vi "Measure DC 120629.vi"() -> ()   [LabVIEW 2011] (continued)
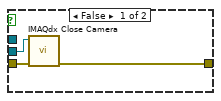
[diagram p3: hidden frame]
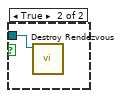
[diagram p7: hidden frame]
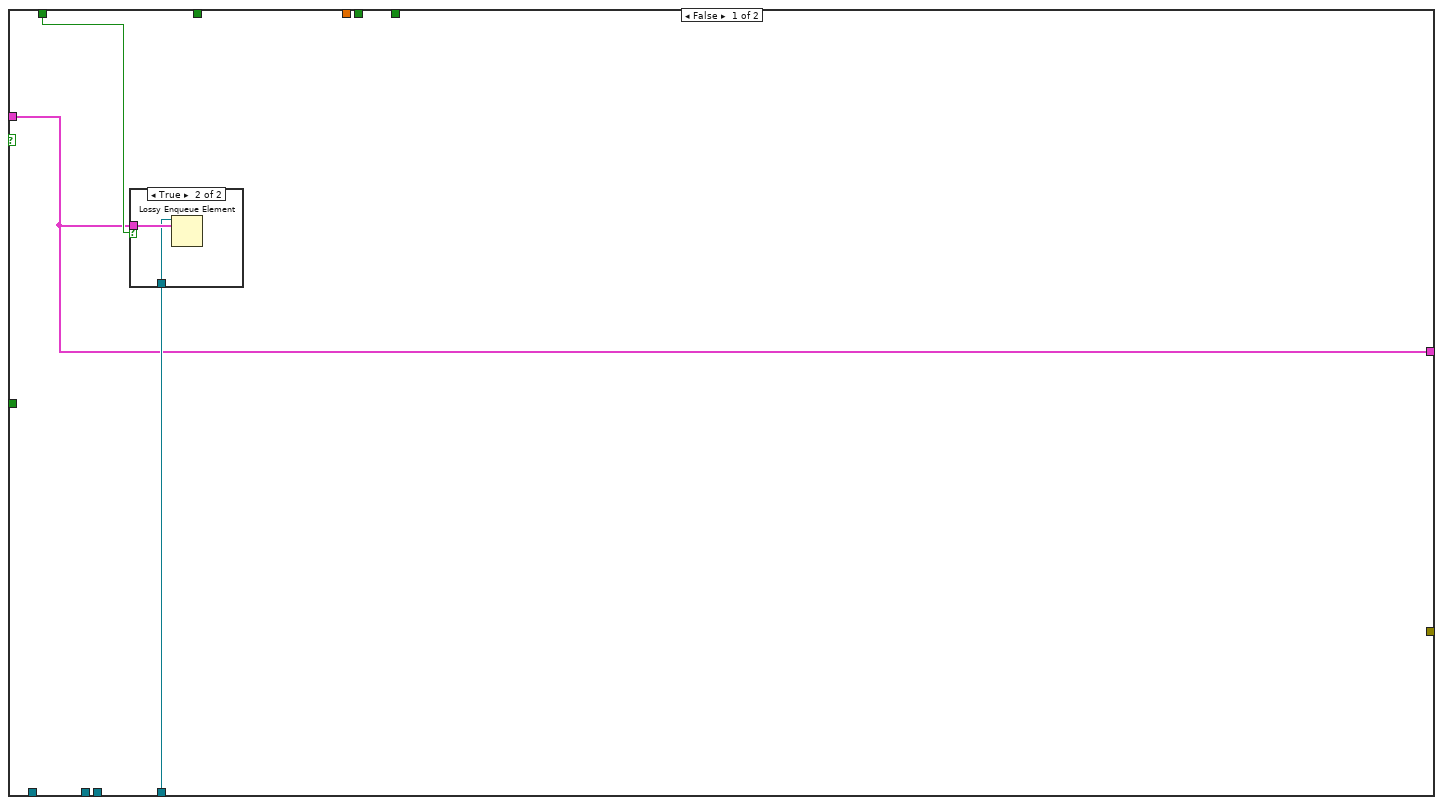
[diagram p10: hidden frame]
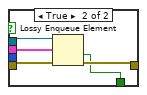
[diagram p13: hidden frame]
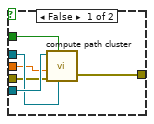
[diagram p17: hidden frame]
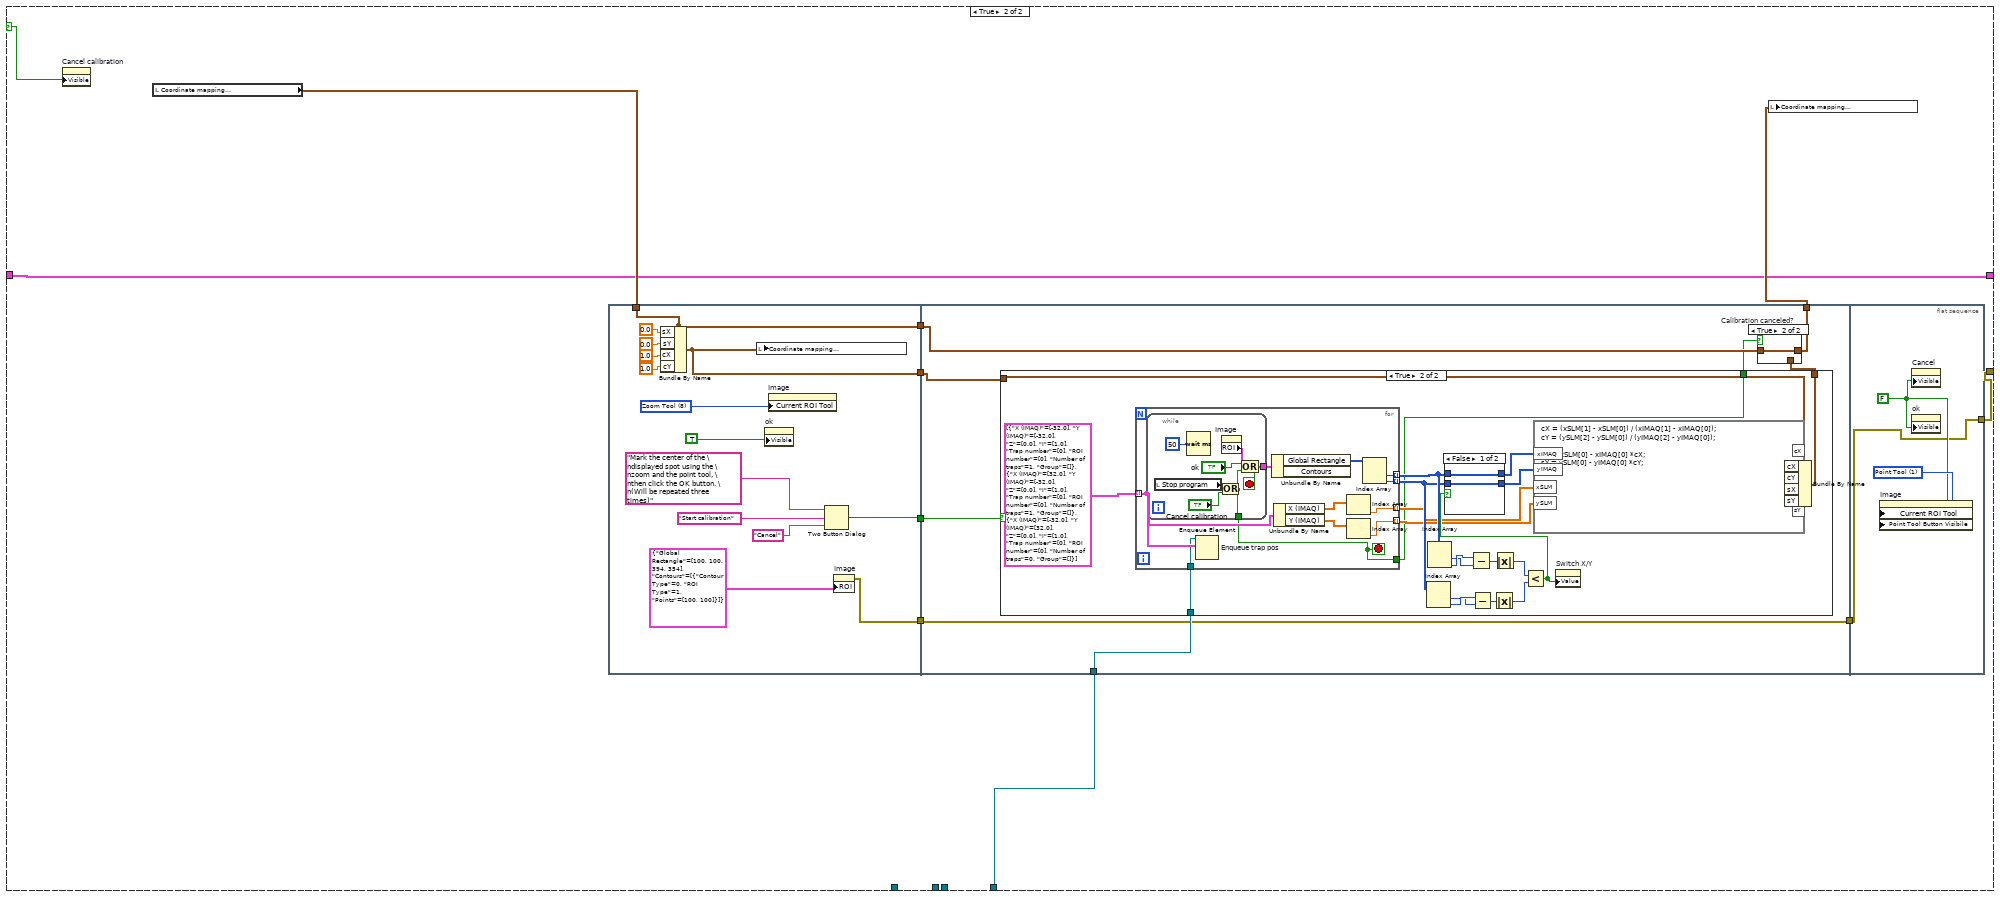
[diagram p18: hidden frame]
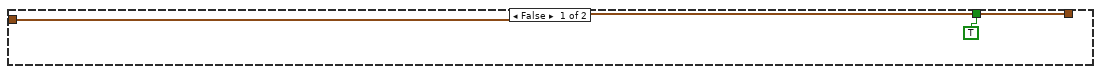
[diagram p20: hidden frame]
        tunnel: w280 -> [_ w301]
        tunnel: w284 -> [_ w300]
        frame False {
        }
        frame True {
          n112 = case shown="True" w305 {
            tunnel: w312 -> [w320 w331]
            tunnel: [w318 w330] -> w310
            tunnel: [w317 w329] -> w309
            tunnel: w311 -> [w318 w328]
            tunnel: [w319 w327] -> w308
            tunnel: [w314 w326] -> w303
            tunnel: [w316 w325] -> w307
            tunnel: w306 -> [w315 w325]
            tunnel: w304 -> [w313 w324]
            tunnel: w302 -> [_ w323]
            tunnel: w301 -> [_ w322]
            tunnel: w300 -> [_ w321]
            frame False {
              n113 = call <vilib>:"IMAQdx Grab.vi"("error in"=w313, "Image In"=w320, "Session In"=w315) -> ("error out"=w317:errorcluster, "Buffer Number Out"=w314:u32, "Image Out"=w319:T2, "Session Out"=w316:T9)  [unwired: 5 in]
            }
            frame True {
              n114 = case shown="True" w323 {
                tunnel: w331 -> [w338 _]
                tunnel: [w337 w346] -> w330
                tunnel: [w336 w348] -> w329
                tunnel: w328 -> [w335 w343]
                tunnel: [w334 w347] -> w327
                tunnel: [w333 w345] -> w326
                tunnel: w324 -> [w332 w344]
                tunnel: w322 -> [_ w340]
                tunnel: w321 -> [_ w339]
                frame False {
                  n115 = call <vilib>:"IMAQ Grab Acquire.vi"("error in (no error)"=w332, "Image In"=w338, "IMAQ Session In"=w335) -> ("error out"=w336:errorcluster, "Acquired Buffer Number"=w333:u32, "Image Out"=w334:T2, "IMAQ Session Out"=w337:refnum<k11>)  [unwired: 1 in, 4 out]
                }
                frame True {
                  n116 = case shown="True" w339 {
                    tunnel: w344 -> [w352 w353]
                    tunnel: w343 -> [w351 _]
                    tunnel: [w350 w353] -> w342
                    tunnel: [w349 w354] -> w341
                    tunnel: w340 -> [_ w354]
                    frame False {
                      n117 = property class="IMAQ"(reference=w351, error in=w352) -> (error out=w350:errorcluster, "Last Valid Frame"=w349:u32)  [unwired: 1 out]
                    }
                    frame True {
                    }
                  }
                  n118 = call <vilib>:"IMAQ Extract Buffer.vi"("error in (no error)"=w342, "Buffer to extract"=w341, "IMAQ Session In"=w343) -> ("error out"=w348:errorcluster, "Buffer Number"=w345:i32, "Image Out"=w347:T2, "IMAQ Session Out"=w346:refnum<k11>)  [unwired: 3 in, 2 out]
                }
              }
            }
          }
        }
      }
      n119 = call "IMAQ Cast Image"("Image Type"=w276, "Image Dst"=w275, "Image Src"=w278) -> ("Image Dst Out"=w273:T2)  [unwired: 7 in, 1 out]
      n120 = call "IMAQ Add"("Image Src A"=w274, "Image Src B"=w273) -> ("Image Dst Out"=w277:T2)  [unwired: 5 in, 1 out]
    }
    n121 = property class="IMAQ"(reference=w235) -> (reference out=w237:refnum<k11>, "Lost Frames"=→"Lost Frames":u32)  [unwired: 1 in, 1 out]
    n122 = call "IMAQ Divide"("Image Src A"=w221, "Constant"="Image\naveraging") -> ("Image Dst Out"=w217:T2)  [unwired: 5 in, 1 out]
    n123 = case shown="False" "?" {
      tunnel: w217 -> [w265 w272]
      tunnel: w216 -> [w264 w271]
      tunnel: [w263 w270] -> w215
      tunnel: "?" -> [w262 _]
      frame False {
        n124 = case shown="True" w262 {
          tunnel: w265 -> [w266 w269]
          tunnel: w264 -> [_ w268]
          tunnel: [w266 w267] -> w263
          frame False {
          }
          frame True {
            n125 = call "IMAQ Subtract"("Image Src A"=w269, "Image Src B"=w268) -> ("Image Dst Out"=w267:T2)  [unwired: 5 in, 1 out]
          }
        }
      }
      frame True {
        n126 = call "IMAQ Copy"("Image Dst"=w271, "Image Src"=w272) -> ("Image Dst Out"=w270:T2)  [unwired: 4 in, 1 out]
      }
    }
    n127 = case shown="True" "?" {
      tunnel: w215 -> [w355 w356]
      tunnel: [w355 w363] -> w228
      tunnel: w209 -> [_ w358]
      frame False {
      }
      frame True {
        w359 = T7 0 items=["Grayscale (U8)", "Grayscale (I16)", "Grayscale (SGL)", "Complex (CSG)", "RGB (U32)", "HSL (U32)", "RGB (U64)", "Grayscale (U16)"] ("Image Type")
        n128 = call "File Dialog"("start path"="start path") -> ("selected path"=w362:path, "cancelled"=w361:bool)  [unwired: 11 in, 2 out]
        n129 = call "IMAQ Cast Image"("Image Type"=w359, "Image Dst"=w358, "Image Src"=w356) -> ("Image Dst Out"=w357:T2)  [unwired: 7 in, 1 out]
        n130 = case shown="False" w361 {
          tunnel: [w364 w367] -> w363
          tunnel: w362 -> [w366 _]
          tunnel: w357 -> [w365 _]
          tunnel: w356 -> [w364 w367]
          frame False {
            n131 = call-poly "IMAQ Write File 2"("File Path"=w366, "Image"=w365) -> ()  [unwired: 8 in, 2 out]
          }
          frame True {
          }
        }
      }
    }
    n132 = call "IMAQ Quantify 2"("Image"=w228) -> ("Global Report"=→"Global Report":T3)  [unwired: 8 in, 2 out]
    n133 = case shown="True" "threshold" {
      tunnel: w228 -> [w368 w375]
      tunnel: [w368 w373] -> w233
      frame False {
      }
      frame True {
        n134 = Unbundle By Name("Range") -> ("Lower value"=w370:sgl)
        n135 = Select(t=w370, s="s", f=sgl 0.0) -> (s? t:f=w378:sgl)
        n136 = Select(t=sgl 0.0 ("Lower value"), s="s", f=w370) -> (s? t:f=w372:sgl)
        n137 = Bundle By Name(cluster="Range", "Lower value"=w372) -> (w376:cluster{"Lower value":sgl, "Upper value":sgl})
        n138 = call "IMAQ Subtract"("Image Src A"=w375, "Constant"=w378) -> ("Image Dst Out"=w374:T2)  [unwired: 5 in, 1 out]
        n139 = call "IMAQ Threshold"("Keep/Replace Value (Replace)"=FALSE, "Range"=w376, "Image Src"=w374) -> ("Image Dst Out"=w373:T2)  [unwired: 7 in, 1 out]
      }
    }
    n140 = case shown="True" "Video tracking" {
      tunnel: w233 -> [w388 w412]
      tunnel: w253 -> [_ w422]
      tunnel: w257 -> [w397 w421]
      tunnel: w245 -> [_ w420]
      tunnel: [w397 w419] -> w244
      tunnel: [_ w418] -> w242
      tunnel: [w381 w398] -> w256
      tunnel: w255 -> [w396 w417]
      tunnel: [w396 w416] -> w241
      tunnel: w248 -> [w393 _]
      tunnel: w249 -> [w392 w414]
      tunnel: "Display path" -> [w390 _]
      tunnel: [w387 w412] -> w232
      tunnel: [FALSE ("timed out?") w410] -> w230
      tunnel: "?" -> [_ w409]
      tunnel: w224 -> [w384 w403]
      tunnel: [w383 w400] -> _
      tunnel: "Switch X/Y" -> [w382 w399]
      tunnel: "ROI size" -> [w381 w398]
      frame False {
        n141 = Get Queue Status(queue=w393, return elements? (F)=w390) -> (elements=w394:T4[])  [unwired: 1 in, 7 out]
        n142 = Preview Queue Element(queue=w392, timeout in ms (-1)=10) -> (element=w391:T4)  [unwired: 1 in, 3 out]
        n143 = call "Create trap overlay.vi"("Current trap cluster"=w391, "Image in"=w388, "ROI size"=w381, "Switch X/Y"=w382, "Path"=w394) -> ("Image Out"=w387:T2)
        n144 = Wait (ms)(milliseconds to wait=u32 100) -> ()  [unwired: 1 out]
        n145 = call <vilib>:"Wait at Rendezvous.vi"("ms timeout (-1)"=0, "rendezvous"=w384) -> ("error out"=w383:errorcluster)  [unwired: 3 in, 2 out]
      }
      frame True {
        n146 = Preview Queue Element(queue=w414) -> (element=w415:T4)  [unwired: 2 in, 3 out]
        n147 = call "Position measurement.vi"("Switch xy"=w399, "ROI size"=w398, "Acquired Buffer Number"=w420, "ROIs"=w422, "Measure \nintensities"=w409, "Trap positions"=w415, "Image"=w412) -> ("Position data out"=w402:T8)  [unwired: 2 in]
        n148 = Enqueue Element(queue=w417, element=w415) -> (queue out=w416:refnum<queue>)  [unwired: 2 in, 2 out]
        n149 = case shown="True" "Display data" {
          tunnel: w402 -> [_ w430]
          frame False {
          }
          frame True {
            n150 = call "Display Cetroids (SubVI).vi"("Measurement data"=w430) -> ()  [unwired: 8 in, 3 out]
          }
        }
        n151 = feedback #1(0) -> (w406:i32)
        n152 = Equal?(x="images per \nhologram", y=w406) -> (x = y?=w404:bool)
        n153 = case shown="True" w404 {
          tunnel: [w424 0] -> w408
          tunnel: w406 -> [w425 _]
          tunnel: w403 -> [_ w428]
          tunnel: w402 -> [w423 w427]
          tunnel: [w423 w427] -> w401
          tunnel: [_ w426] -> w400
          frame False {
            n154 = Increment(x=w425) -> (x+1=w424:i32)
          }
          frame True {
            n155 = call <vilib>:"Wait at Rendezvous.vi"("rendezvous"=w428) -> ("error out"=w426:errorcluster)  [unwired: 4 in, 2 out]
          }
        }
        n156 = feedback-in #1(w408) -> ()
        n157 = Enqueue Element(queue=w421, element=w401, timeout in ms (-1)=10000) -> (queue out=w419:refnum<queue>, timed out?=w410:bool, error out=w418:errorcluster)  [unwired: 1 in]
      }
    }
    n158 = Or(x="Save data", y=w230) -> (x .or. y?=w231:bool)
    n159 = case shown="True" "?" {
      tunnel: w232 -> [_ w454]
      frame False {
      }
      frame True {
        "Image" <- w454
      }
    }
    n160 = case shown="True" w231 {
      tunnel: w244 -> [w432 w439]
      tunnel: w242 -> [_ w442]
      tunnel: w241 -> [w431 w440]
      frame False {
        n161 = case shown="False" "Purge data" {
          tunnel: w432 -> [_ w435]
          tunnel: w431 -> [_ w434]
          frame False {
          }
          frame True {
            n162 = Flush Queue(queue=w435) -> ()  [unwired: 1 in, 3 out]
            n163 = Flush Queue(queue=w434) -> ()  [unwired: 1 in, 3 out]
          }
        }
      }
      frame True {
        n164 = Flush Queue(queue=w439, error in (no error)=w442) -> (remaining elements=w438:T14)  [unwired: 2 out]
        n165 = Flush Queue(queue=w440, error in (no error)=w442) -> (remaining elements=w437:T4[])  [unwired: 2 out]
        n166 = for {
          tunnel: w438 -> [w453] mode=indexing
          tunnel: w437 -> [w452] mode=indexing
          workers-P: _ -> [_]
          tunnel: [w451] -> w441 mode=indexing
          n167 = Bundle("output cluster 2"=w453, "output cluster 2"=w452) -> (w451:T15)  [unwired: 1 in]
        }
        n168 = Write to Binary File(data=w441) -> (cancelled=w436:bool)  [unwired: 5 in, 2 out]
        n169 = case shown="True" w436 {
          tunnel: w440 -> [_ w446]
          tunnel: w439 -> [_ w445]
          tunnel: w438 -> [_ w444]
          tunnel: w437 -> [_ w443]
          frame False {
          }
          frame True {
            n170 = for {
              tunnel: w446 -> [w450]
              tunnel: w445 -> [w449]
              tunnel: w444 -> [w448] mode=indexing
              tunnel: w443 -> [w447] mode=indexing
              n171 = Enqueue Element(queue=w449, element=w448) -> ()  [unwired: 2 in, 3 out]
              n172 = Enqueue Element(queue=w450, element=w447) -> ()  [unwired: 2 in, 3 out]
            }
          }
        }
      }
    }
    n173 = local read "Stop program"() -> (w258:bool)
  }
  n174 = property class="Bool (strict)"("Visible"=w49) -> ()  [unwired: 2 in, 2 out]
  n175 = property on="ROI size" class="DigNum (strict)"("Visible"=w49) -> ()  [unwired: 2 in, 2 out]
  n176 = property on="Video tracking" class="Bool (strict)"("Visible"=w49) -> ()  [unwired: 2 in, 2 out]
  n177 = property on="Save data" class="Bool"("Visible"=w49) -> ()  [unwired: 2 in, 2 out]
  n178 = property on="Purge data" class="Bool"("Visible"=w49) -> ()  [unwired: 2 in, 2 out]
  n179 = call "FreeGPUandSLM.vi"("error in"=w14) -> ("error out"=w46:errorcluster)  [unwired: 1 out]
  "CUDA/SLM error" <- w46
  n180 = call-poly <vilib>:"Close Input Device.vi"("error in (no error)"=w42, "device ID"=w44) -> ()  [unwired: 9 out]
  n181 = while "Trap position loop" {
    tunnel: w29 -> [w464]
    tunnel: w30 -> [w461]
    shift-right: [w463] -> _
    shift-left: w27 -> [w458]
    tunnel: w19 -> [w462]
    tunnel: w28 -> [w460]
    tunnel: w36 -> [_]
    tunnel: [w457] -> w47
    tunnel: w11 -> [w456]
    stop <- "Stop program" stop-if-true
    n182 = case shown="False" "Run calibration" {
      selector: "Run calibration" -> [_ w606]
      tunnel: w464 -> [w487 _]
      tunnel: w458 -> [w486 w605]
      tunnel: [w469 w605] -> w463
      tunnel: w462 -> [w476 w613]
      tunnel: w461 -> [w474 _]
      tunnel: w460 -> [w471 _]
      tunnel: [w466 w607] -> w457
      frame False {
        n183 = case "Update trap cluster" shown="True" "Edit trap cluster" {
          tunnel: w486 -> [w488 w493]
          tunnel: [w488 w492] -> w477
          frame False {
          }
          frame True {
            n184 = local read "Coordinate mapping \n(IMAQ to SLM)"() -> (w490:T6)
            n185 = call "Edit trap cluster.vi"("Coordinate mapping \n(IMAQ to SLM)"=w490, "trap cluster in"=w493) -> ("SubVI closed"=w491:bool, "Trap cluster out"=w492:T4)
            n186 = Not(x=w491) -> (.not. x?=w489:bool)
            n187 = local write "Edit trap cluster"(w489) -> ()
          }
        }
        n188 = Wait (ms)(milliseconds to wait=u32 50) -> ()  [unwired: 1 out]
        n189 = Unbundle By Name("Path controls") -> ("Add current \npositions to path"=w472:bool, "Synchronize traps"=w481:bool, "Step length"=w484:dbl, "follow path"=w475:bool, "Arrive \nsimultaneously"=w483:bool)
        n190 = Or(x=w472, y=w481) -> (x .or. y?=w482:bool)
        n191 = Or(x=w481, y=w475) -> (x .or. y?=w479:bool)
        n192 = Or(x=w482, y=w475) -> (x .or. y?=w480:bool)
        n193 = case shown="True" "Create path" {
          tunnel: w487 -> [_ w503]
          tunnel: w477 -> [w494 w500]
          tunnel: w484 -> [_ w512]
          tunnel: w474 -> [_ w507]
          tunnel: w483 -> [_ w511]
          tunnel: w480 -> [_ w510]
          tunnel: w479 -> [_ w509]
          tunnel: w475 -> [_ w508]
          tunnel: w476 -> [w496 w504]
          tunnel: w471 -> [_ w502]
          tunnel: "Updating trap cluster" -> [w495 _]
          tunnel: [w494 w501] -> w469
          tunnel: [_ w499] -> w466
          frame False {
            n194 = case shown="True" w495 {
              tunnel: w494 -> [_ w498]
              tunnel: w496 -> [_ w497]
              frame False {
              }
              frame True {
                n195 = Lossy Enqueue Element(queue=w497, element=w498) -> ()  [unwired: 1 in, 4 out]
              }
            }
          }
          frame True {
            n196 = Lossy Enqueue Element "Enqueue\noverlay pos"(queue=w502, element=w500) -> ()  [unwired: 1 in, 4 out]
            n197 = case "Add wpt" shown="True" w510 {
              tunnel: w500 -> [_ w585]
              tunnel: w503 -> [w582 w586]
              tunnel: [w582 w583] -> w513
              tunnel: [_ w584] -> w505
              frame False {
              }
              frame True {
                n198 = Enqueue Element "Enqueue path\n waypts"(queue=w586, element=w585) -> (queue out=w583:refnum<queue>, error out=w584:errorcluster)  [unwired: 2 in, 1 out]
              }
            }
            n199 = case "Compute path" shown="True" w509 {
              tunnel: w513 -> [_ w593]
              tunnel: w507 -> [_ w592]
              tunnel: w512 -> [_ w591]
              tunnel: w511 -> [_ w589]
              tunnel: [w587 w588] -> w506
              tunnel: w505 -> [w587 w590]
              frame False {
              }
              frame True {
                n200 = case shown="True" "Intensity path" {
                  tunnel: w593 -> [w600 w604]
                  tunnel: w592 -> [w599 w603]
                  tunnel: w591 -> [w598 _]
                  tunnel: w590 -> [w597 w601]
                  tunnel: w589 -> [w596 _]
                  tunnel: [w595 w601] -> w588
                  frame False {
                    n201 = call "compute path cluster.vi"("path queue"=w599, "Arrive simultaeously"=w596, "error in (no error)"=w597, "Step length\n(IMAQ pixels)"=w598, "waypoint queue"=w600) -> ("error out"=w595:errorcluster)  [unwired: 2 in]
                  }
                  frame True {
                    n202 = call "Compute I path (SubVI).vi"("I step"="I step", "wpt"=w604, "Path"=w603) -> ()  [unwired: 9 in]
                  }
                }
              }
            }
            n203 = case "Follow path" shown="True" w508 {
              tunnel: w507 -> [_ w537]
              tunnel: w506 -> [_ w538]
              tunnel: w504 -> [_ w540]
              tunnel: w503 -> [_ w539]
              tunnel: [w514 w517] -> w501
              tunnel: w500 -> [w514 _]
              tunnel: [_ w515] -> w499
              frame False {
              }
              frame True {
                w533 = TRUE ("Visible")
                n204 = local write "Display path"(FALSE ("Display path")) -> ()
                n205 = Flush Queue "Flush Waypts"(queue=w539, error in (no error)=w538) -> (error out=w532:errorcluster)  [unwired: 2 out]
                n206 = Get Queue Status(queue=w537, error in (no error)=w532) -> (queue out=w536:refnum<queue>, error out=w531:errorcluster, # elements in queue=w535:i32)  [unwired: 1 in, 5 out]
                n207 = property on="Pause" class="Bool (strict)"(error in=w531, "Visible"=w533) -> (error out=w530:errorcluster)  [unwired: 1 in, 1 out]
                n208 = property on="cancel path" class="Bool"(error in=w530, "Visible"=w533) -> (error out=w529:errorcluster)  [unwired: 1 in, 1 out]
                n209 = for {
                  N: w535 -> [_]
                  tunnel: w529 -> [w559]
                  tunnel: w540 -> [w561]
                  tunnel: w536 -> [w557]
                  tunnel: [w557] -> w534
                  tunnel: [FALSE ("Group traps")] -> w516
                  shift-right: [w548] -> w517
                  shift-left: _ -> [w550]
                  tunnel: [w547] -> w528
                  tunnel: [w544] -> w526 mode=indexing
                  tunnel: [w545] -> w522
                  tunnel: [TRUE ("Display path")] -> w520
                  i -> [w545]
                  stop <- w554 stop-if-true
                  n210 = Dequeue Element(queue=w557, timeout in ms (-1)=0, error in (no error)=w559) -> (element=w549:T4, timed out?=w553:bool, error out=w560:errorcluster)  [unwired: 1 out]
                  n211 = while {
                    tunnel: [w579] -> w551
                    tunnel: ["cancel path"] -> w546
                    stop <- w581 stop-if-true
                    n212 = local read "Stop program"() -> (w579:bool)
                    n213 = Wait (ms)(milliseconds to wait="Step time \n(ms)") -> ()  [unwired: 1 out]
                    n214 = Or(x=w579, y="cancel path") -> (x .or. y?=w577:bool)
                    n215 = Implies(1:w577, 2:"Pause") -> (0:w581:bool)
                  }
                  n216 = case shown="False" "Skip step if \ntimed out" {
                    tunnel: w561 -> [w568 w573]
                    tunnel: w560 -> [w567 w571]
                    tunnel: [FALSE ("overflow?") w569] -> w552
                    tunnel: w549 -> [w566 w572]
                    tunnel: [w565 w570] -> w547
                    tunnel: 500 ("timeout in ms (-1)") -> [w564 _]
                    frame False {
                      n217 = Enqueue Element "Enqueue trap pos"(queue=w568, element=w566, timeout in ms (-1)=w564, error in (no error)=w567) -> (timed out?=→"timed out?":bool, error out=w565:errorcluster)  [unwired: 1 out]
                    }
                    frame True {
                      n218 = Lossy Enqueue Element(queue=w573, element=w572, error in (no error)=w571) -> (overflow?=w569:bool, error out=w570:errorcluster)  [unwired: 2 out]
                    }
                  }
                  "Step skipped" <- w552
                  n219 = case shown="False" w551 {
                    tunnel: w550 -> [_ w575]
                    tunnel: w549 -> [w574 _]
                    tunnel: [w574 w575] -> w548
                    frame False {
                    }
                    frame True {
                    }
                  }
                  n220 = Or(x=w546, y=w551) -> (x .or. y?=w556:bool)
                  n221 = Or(x=w556, y=w553) -> (x .or. y?=w554:bool)
                  n222 = Tick Count (ms)() -> (millisecond timer value=w544:u32)
                }
                n223 = local write "Step skipped"(w516) -> ()
                n224 = local write "Create path"(w516) -> ()
                n225 = local write "Display path"(w520) -> ()
                n226 = property on="follow path" class="Bool (strict)"("Value"=w516) -> ()  [unwired: 2 in, 2 out]
                n227 = property on="Pause" class="Bool (strict)"(error in=w528, "Visible"=w516, "Value"=w516) -> (error out=w527:errorcluster)  [unwired: 1 in, 1 out]
                n228 = Array Max & Min(array=w526) -> (max value=w525:u32, min value=w524:u32)  [unwired: 2 out]
                n229 = Subtract(x=w525, y=w524) -> (x-y=w523:u32)
                n230 = Increment(x=w522) -> (x+1=w519:i32)
                n231 = property on="cancel path" class="Bool"(error in=w527, "Visible"=w516) -> (error out=w515:errorcluster)  [unwired: 1 in, 1 out]
                n232 = Divide(x=w523, y=w519) -> (x/y=→"Average step time (ms)":dbl)
                n233 = Flush Queue "Flush Path"(queue=w534) -> ()  [unwired: 1 in, 3 out]
              }
            }
          }
        }
        n234 = case shown="True" "Apply Corrections" {
          frame False {
          }
          frame True {
            n235 = call "Apply Corrections.vi"() -> ()  [unwired: 1 in]
          }
        }
      }
      frame True {
        n236 = property on="Cancel calibration" class="Bool"("Visible"=w606) -> ()  [unwired: 2 in, 2 out]
        n237 = local read "Coordinate mapping \n(IMAQ to SLM)"() -> (w612:T6)
        n238 = flat-sequence {
          tunnel: [w625] -> w615
          tunnel: w612 -> [w618]
          tunnel: [w616] -> w611
          tunnel: [w618] -> w610
          tunnel: [w617] -> w608
          tunnel: w615 -> [w632]
          tunnel: [w634] -> w614
          tunnel: w613 -> [w637]
          tunnel: w611 -> [w636]
          tunnel: w610 -> [w633]
          tunnel: [w630] -> w609
          tunnel: w608 -> [w630]
          tunnel: w609 -> [w688]
          tunnel: [w688] -> w607
          frame #0 {
            w626 = u32 8 items=["Zoom Tool"=8, "Selection Tool"=0, "Pan Tool"=9, "Point Tool"=1, "Line Tool"=2, "Rectangle Tool"=3, "Rotated Rectangle Tool"=12, "Polyline Tool"=10, "Polygon Tool"=5, "Freehand Tool"=11, "Closed Freehand Tool"=6, "Ellipse Tool"=4, "Annulus Tool"=7] ("Current ROI Tool")
            n239 = Bundle By Name(cluster=w618, "sX"=0.0, "sY"=0.0, "cX"=1.0 ("sX"), "cY"=1.0) -> (w616:T6)
            n240 = local write "Coordinate mapping \n(IMAQ to SLM)"(w616) -> ()
            n241 = property on="ok" class="Bool"("Visible"=TRUE ("ROI Tool Buttons Visibile:Zoom Tool Button Visible")) -> ()  [unwired: 2 in, 2 out]
            n242 = property on="Image" class="ImageControl"("Current ROI Tool"=w626) -> ()  [unwired: 2 in, 2 out]
            n243 = Two Button Dialog(message="Mark the center of the \ndisplayed spot using the \nzoom and the point tool, \nthen click the OK button. \n(Will be repeated three times)", 1:"Cancel" ("F button name (\"Cancel\")"), 2:"Start calibration" ("T button name (\"OK\")")) -> (T button?=w625:bool)
            n244 = property on="Image" class="ImageControl"("ROI"=T1 {"Global Rectangle"=[100, 100, 394, 354], "Contours"=[{"Contour Type"=0, "ROI Type"=1, "Points"=[100, 100]}]} ("ROI 2")) -> (error out=w617:errorcluster)  [unwired: 2 in, 1 out]
          }
          frame #1 {
            n245 = case shown="True" w632 {
              tunnel: w636 -> [w641 w652]
              tunnel: [w641 w647] -> w635
              tunnel: w637 -> [_ w643]
              tunnel: [TRUE ("Stop program") w642] -> w631
              frame False {
              }
              frame True {
                n246 = for {
                  tunnel: [w679] -> w661 mode=indexing
                  tunnel: [w678] -> w660 mode=indexing
                  tunnel: T4[] [{"X (IMAQ)"=[-32.0], "Y (IMAQ)"=[-32.0], "Z"=[0.0], "I"=[1.0], "Trap number"=[0], "ROI number"=[0], "Number of traps"=1, "Group"=[]}, {"X (IMAQ)"=[32.0], "Y (IMAQ)"=[-32.0], "Z"=[0.0], "I"=[1.0], "Trap number"=[0], "ROI number"=[0], "Number of traps"=1, "Group"=[]}, {"X (IMAQ)"=[-32.0], "Y (IMAQ)"=[32.0], "Z"=[0.0], "I"=[1.0], "Trap number"=[0], "ROI number"=[0], "Number of traps"=0, "Group"=[]}] -> [w676] mode=indexing
                  tunnel: [w673] -> w645 mode=indexing
                  tunnel: [w671] -> w644 mode=indexing
                  tunnel: w643 -> [w675]
                  tunnel: [w670] -> w642
                  stop <- w670 stop-if-true
                  n247 = while {
                    tunnel: [w686] -> w677
                    tunnel: [w682] -> w670
                    stop <- w684 stop-if-true
                    n248 = local read "Stop program"() -> (w683:bool)
                    n249 = Wait (ms)(milliseconds to wait=u32 50) -> ()  [unwired: 1 out]
                    n250 = Or(x=w683, y="Cancel calibration") -> (x .or. y?=w682:bool)
                    n251 = property on="Image" class="ImageControl"() -> ("ROI"=w686:T1)  [unwired: 2 in, 2 out]
                    n252 = Or(x="ok", y=w682) -> (x .or. y?=w684:bool)
                  }
                  n253 = Enqueue Element "Enqueue trap pos"(queue=w675, element=w676) -> ()  [unwired: 2 in, 3 out]
                  n254 = Unbundle By Name(w677) -> ("Global Rectangle"=w680:i32[])  [unwired: 1 out]
                  n255 = Unbundle By Name(w676) -> ("X (IMAQ)"=w674:sgl[], "Y (IMAQ)"=w672:sgl[])
                  n256 = Index Array(array=w674) -> (element=w673:sgl)  [unwired: 1 in]
                  n257 = Index Array(array=w672) -> (element=w671:sgl)  [unwired: 1 in]
                  n258 = Index Array(array=w680) -> (element #1=w679:i32, element #2=w678:i32)  [unwired: 2 in]
                }
                n259 = Index Array(array=w660) -> (element #1=w662:i32, element #2=w663:i32)  [unwired: 2 in]
                n260 = Index Array(array=w661) -> (element #1=w664:i32, element #2=w665:i32)  [unwired: 2 in]
                n261 = Subtract(x=w665, y=w664) -> (x-y=w657:i32)
                n262 = Subtract(x=w663, y=w662) -> (x-y=w655:i32)
                n263 = Absolute Value(x=w655) -> (abs(x)=w654:i32)
                n264 = Absolute Value(x=w657) -> (abs(x)=w656:i32)
                n265 = Less?(x=w656, y=w654) -> (x < y?=w653:bool)
                n266 = case shown="False" w653 {
                  tunnel: w661 -> [w667 w669]
                  tunnel: w660 -> [w666 w668]
                  tunnel: [w666 w669] -> w658
                  tunnel: [w667 w668] -> w659
                  frame False {
                  }
                  frame True {
                  }
                }
                n267 = formula code="cX = (xSLM[1] - xSLM[0]) / (xIMAQ[1] - xIMAQ[0]); \ncY = (ySLM[2] - ySLM[0]) / (yIMAQ[2] - yIMAQ[0]); \n\nsX = xSLM[0] - xIMAQ[0] *cX;\nsY = ySLM[0] - yIMAQ[0] *cY;"("xIMAQ"=w659, "yIMAQ"=w658, "xSLM"=w645, "ySLM"=w644) -> ("cX"=w651:dbl, "cY"=w650:dbl, "sX"=w649:dbl, "sY"=w648:dbl)
                n268 = property on="Switch X/Y" class="Bool (strict)"("Value"=w653) -> ()  [unwired: 2 in, 2 out]
                n269 = Bundle By Name(cluster=w652, "cX"=w651, "cY"=w650, "sX"=w649, "sY"=w648) -> (w647:T6)
              }
            }
            n270 = case "Calibration canceled?" shown="True" w631 {
              tunnel: w635 -> [w638 _]
              tunnel: [w638 w639] -> w634
              tunnel: w633 -> [_ w639]
              frame False {
              }
              frame True {
              }
            }
          }
          frame #2 {
            w689 = FALSE ("ROI Tool Buttons Visibile:Zoom Tool Button Visible")
            w690 = u32 1 items=["Zoom Tool"=8, "Selection Tool"=0, "Pan Tool"=9, "Point Tool"=1, "Line Tool"=2, "Rectangle Tool"=3, "Rotated Rectangle Tool"=12, "Polyline Tool"=10, "Polygon Tool"=5, "Freehand Tool"=11, "Closed Freehand Tool"=6, "Ellipse Tool"=4, "Annulus Tool"=7] ("Current ROI Tool")
            n271 = property on="Image" class="ImageControl"("Current ROI Tool"=w690, "Point Tool Button Visibile"=w689) -> ()  [unwired: 2 in, 2 out]
            n272 = property on="Cancel" class="Bool"("Visible"=w689) -> ()  [unwired: 2 in, 2 out]
            n273 = property on="ok" class="Bool"("Visible"=w689) -> ()  [unwired: 2 in, 2 out]
          }
        }
        n274 = local write "Coordinate mapping \n(IMAQ to SLM)"(w614) -> ()
      }
    }
    n275 = case shown="False" "Stop program" {
      tunnel: w456 -> [_ w465]
      frame False {
      }
      frame True {
        n276 = call <vilib>:"Destroy Rendezvous.vi"("rendezvous"=w465) -> ()  [unwired: 5 in, 2 out]
      }
    }
  }
  n277 = for {
    tunnel: w52 -> [w691] mode=indexing
    n278 = call "IMAQ Dispose"("Image"=w691) -> ()  [unwired: 5 in, 1 out]
  }
  n279 = case shown="True" w31 {
    tunnel: w60 -> [_ w697]
    tunnel: w59 -> [w692 w696]
    tunnel: w50 -> [_ w695]
    tunnel: w33 -> [_ w694]
    tunnel: [w692 w693] -> w48
    frame False {
    }
    frame True {
      n280 = case shown="True" w694 {
        tunnel: w697 -> [_ w703]
        tunnel: w696 -> [w700 w702]
        tunnel: [w699 w701] -> w693
        tunnel: w695 -> [w698 _]
        frame False {
          n281 = call <vilib>:"IMAQdx Close Camera.vi"("error in"=w700, "Session In"=w698) -> ("error out"=w699:errorcluster)  [unwired: 9 in]
        }
        frame True {
          n282 = call <vilib>:"IMAQ Close.vi"("error in (no error)"=w702, "IMAQ Session In"=w703) -> ("error out"=w701:errorcluster)  [unwired: 9 in]
        }
      }
    }
  }
  n283 = Merge Errors(w48, w47) -> (w45:errorcluster)
  "NI Vision error" <- w45
  n284 = call "IMAQ Dispose"("Image"=w51) -> ()  [unwired: 5 in, 1 out]
  n285 = flat-sequence {
    tunnel: w46 -> [_]
    tunnel: w45 -> [_]
    frame #0 {
      n286 = local write "Stop program"(FALSE ("Stop program")) -> ()
    }
  }
